vi "UHR-Fleezers Control (host) - 10.6.vi"() -> ()   [LabVIEW 2010] (continued)
            n291 = xnode "Read/Write Control"("FPGA VI Reference In"=w3084, "error in"=w3083, "AI to FIFO"=w3087, "APD to FIFO"=w3087, "Start scan"=w3087, "Start scan (MCL)"=w3087) -> ("FPGA VI Reference Out"=w3089:T20, "error out"=w3088:errorcluster)
          }
        }
        "Raster Scanning..." <- TRUE ("Scanning...")
      }
    }
    n292 = And(x="Save scans", y=w1186) -> (x .and. y?=w1230:bool)
    n293 = Compound Arithmetic op=OR("Start MCL Scan", "Confocal Image", "Confocal Linescan") -> (w1184:bool)
    n294 = And(x="Save Data (MCL)", y=w1184) -> (x .and. y?=w1229:bool)
    n295 = case "Start MCL raster scan" shown="False" w1184 {
      tunnel: w1232 -> [w2240 w2255]
      tunnel: w1231 -> [w2239 w2254]
      tunnel: [w2240 w2250] -> w991
      tunnel: [w2239 w2249] -> w990
      tunnel: [FALSE w2248] -> w1215
      tunnel: "Start MCL Scan" -> [_ w2243]
      tunnel: "Confocal Image" -> [_ w2242]
      tunnel: "Confocal Linescan" -> [_ _]
      frame False {
      }
      frame True {
        w2248 = TRUE
        n296 = case shown="True" "Restart DMA? (MCL)" {
          tunnel: [w2500 w2502] -> w2253
          tunnel: [w2499 w2501] -> w2252
          tunnel: w2255 -> [w2500 w2505]
          tunnel: w2254 -> [w2499 w2504]
          frame False {
          }
          frame True {
            n297 = call "reset FPGA DMA.vi"("error in"=w2504, "FPGA VI Reference In"=w2505) -> ("error out"=w2501:errorcluster, "FPGA VI Reference Out"=w2502:T20)
            n298 = local write "Overflow (data lost)"(FALSE ("Overflow (data lost)")) -> ()
          }
        }
        n299 = case shown="False" w2243 {
          selector: w2243 -> [_ w2259]
          tunnel: w2242 -> [w2258 _]
          tunnel: [w2258 w2259] -> w2241
          frame False {
            n300 = property on="2D or 1D Scan" class="Bool (strict)"("Val(Sgnl)"=w2258) -> ()  [unwired: 2 in, 2 out]
            n301 = property on="Confocal Image" class="Bool (strict)"("Value"=FALSE ("Start Confocal Map")) -> ()  [unwired: 2 in, 2 out]
          }
          frame True {
          }
        }
        n302 = local write "MCL Scanning"(w2248) -> ()
        n303 = local read "AO1"() -> (w2245:dbl)
        n304 = local read "AO2"() -> (w2244:dbl)
        n305 = case shown="True" "Center Scan" {
          tunnel: w2253 -> [w2266 w2378]
          tunnel: w2252 -> [w2265 w2377]
          tunnel: [w2264 w2376] -> w2250
          tunnel: [w2263 w2375] -> w2249
          tunnel: [w2261 w2362] -> w2247
          tunnel: [w2260 w2361] -> w2246
          tunnel: w2245 -> [w2261 w2367]
          tunnel: w2244 -> [w2260 w2370]
          tunnel: w2241 -> [_ _]
          frame False {
            w2262 = TRUE ("AI to FIFO")
            n306 = xnode "Read/Write Control"("FPGA VI Reference In"=w2266, "error in"=w2265, "AI to FIFO"=w2262, "APD to FIFO"=w2262, "Start scan (MCL)"=w2262) -> ("FPGA VI Reference Out"=w2264:T20, "error out"=w2263:errorcluster)
          }
          frame True {
            w2374 = TRUE ("AI to FIFO")
            n307 = local read "Scan steps (MCL)"() -> (w2353:u64)
            n308 = local read "Scan lines (y)"() -> (w2349:u64)
            n309 = local read "Fast Scan Dir"() -> (w2360:bool)
            n310 = local read "Actual MCL Inc (V)"() -> (w2350:dbl)
            n311 = Decrement(x=w2349) -> (x-1=w2348:u64)
            n312 = Decrement(x=w2353) -> (x-1=w2352:u64)
            n313 = Multiply(x=w2350, y=w2348) -> (x*y=w2347:dbl)
            n314 = Divide(x=w2347, y=2.0) -> (x/y=w2357:dbl)
            n315 = Multiply(x=w2350, y=w2352) -> (x*y=w2351:dbl)
            n316 = Divide(x=w2351, y=2.0) -> (x/y=w2356:dbl)
            n317 = Select(t=w2356, s=w2360, f=w2357) -> (s? t:f=w2355:dbl)
            n318 = Select(t=w2357, s=w2360, f=w2356) -> (s? t:f=w2359:dbl)
            n319 = Subtract(x=w2367, y=w2359) -> (x-y=w2358:dbl)
            n320 = Subtract(x=w2370, y=w2355) -> (x-y=w2354:dbl)
            n321 = local read "2D or 1D Scan"() -> (w2372:bool)
            n322 = Not(x=w2360) -> (.not. x?=w2366:bool)
            n323 = Not(x=w2372) -> (.not. x?=w2368:bool)
            n324 = And(x=w2360, y=w2368) -> (x .and. y?=w2369:bool)
            n325 = And(x=w2368, y=w2366) -> (x .and. y?=w2371:bool)
            n326 = Select(t=w2370, s=w2371, f=w2354) -> (s? t:f=w2361:dbl)
            n327 = Select(t=w2367, s=w2369, f=w2358) -> (s? t:f=w2362:dbl)
            n328 = call "Volt to I16.vi"("Voltage In"=w2362) -> ("I16 Voltage Out"=w2365:i16)
            n329 = call "Volt to I16.vi"("Voltage In"=w2361) -> ("I16 Voltage Out"=w2364:i16)
            n330 = xnode "Read/Write Control"("FPGA VI Reference In"=w2378, "error in"=w2377, "AI to FIFO"=w2374, "APD to FIFO"=w2374, "Start scan (MCL)"=w2374, "AO1"=w2365, "AO2"=w2364) -> ("FPGA VI Reference Out"=w2376:T20, "error out"=w2375:errorcluster)
          }
        }
        "Initial Y" <- w2247
        "Initial X" <- w2246
        "wait to reset values" <- w2248
      }
    }
    n331 = local read "Trap Pos Elements/DMA read"() -> (w1065:u32)
    n332 = local read "Trap AI Elements/DMA read"() -> (w989:u32)
    n333 = local read "APD Elements/DMA read"() -> (w1108:u32)
    n334 = local read "Trap AI FIFO Depth"() -> (w1279:u32)
    n335 = xnode "Invoke Method"("FPGA VI Reference In"=w991, "error in"=w990, "Number of Elements"=w1065, "Timeout (ms)"=-1) -> ("Data"=w1029:u16[], "Elements Remaining"=→"Trap Pos FIFO El Remaining":u32)  [unwired: 2 out]
    n336 = xnode "Invoke Method"("FPGA VI Reference In"=w991, "error in"=w990, "Number of Elements"=w989, "Timeout (ms)"=-1 ("Timeout")) -> ("FPGA VI Reference Out"=w993:T20, "error out"=w992:errorcluster, "Data"=w988:i16[], "Elements Remaining"=w994:u32)
    "Trap AI FIFO El. Rem." <- w994
    n337 = xnode "Get APD Data"("FPGA VI Reference In"=w991, "error in"=w990, "Number of Elements"=w1108, "Timeout (ms)"=-1) -> ("Data"=w1107:u32[], "Elements Remaining"=→"APD FIFO Elements Remaining":u32)  [unwired: 2 out]
    n338 = Subtract(x=w1279, y=w989) -> (x-y=w1278:u32)
    n339 = Decimate 1D Array(w1029) -> (w1026:u16[], w1028:u16[], w1027:u16[])
    n340 = Divide(x=w994, y=w1278) -> (x/y=w1277:dbl)
    "Buffer Status" <- w1277
    n341 = To Unsigned Long Integer(number=w1026) -> (unsigned 32bit integer=w1025:u32[])
    n342 = Join Numbers(hi=w1028, lo=w1027) -> ((hi.lo)=w1024:u32[])
    n343 = Equal?(x=w1277, y=1.0) -> (x = y?=w1275:bool)
    n344 = Join Numbers(hi=w1025, lo=w1024) -> ((hi.lo)=w1018:u64[])
    n345 = call "IR AOM word to freq - vec.vi"("Frequency Word In (double vec)"=w1018) -> ("Frequency Out"=w1064:dbl[])
    n346 = case "Alert buffer overflow" shown="True" w1275 {
      frame False {
      }
      frame True {
        n347 = call <vilib>:"Beep.vi"() -> ()  [unwired: 3 in, 9 out]
        "Overflow (data lost)" <- TRUE ("Overflow (data lost)")
      }
    }
    n348 = Decimate 1D Array(w1064) -> (w1063:dbl[], w1062:dbl[])
    n349 = Array Size(array=w988) -> (size(s)=→"Waveform Chart":i32)
    n350 = Build Array(w1063, w1062) -> (w1061:dbl[][])
    n351 = local read "Trap Sets"() -> (w1145:u32)
    n352 = case "Deinterlace trap data, average down PSD" shown="2" w1145 {
      tunnel: w988 -> [w2535 w2600]
      tunnel: [w2532 w2597] -> w1138
      tunnel: [w2535 w2599] -> w1021
      tunnel: "Detector Type" -> [w2534 w2595]
      tunnel: [w2533 w2598] -> w1137
      tunnel: [w2531 w2596] -> w1250
      frame 1, Default {
        n353 = Divide(x=w2535, y=3276.7) -> (x/y=w2536:dbl[])
        n354 = Decimate 1D Array(w2536) -> (w2545:dbl[], w2544:dbl[], w2543:dbl[], w2542:dbl[], w2541:dbl[], w2540:dbl[], w2539:dbl[], w2538:dbl[])
        n355 = case shown="\"IR-QPD + PSD + FB-QPD position\"" w2534 {
          tunnel: w2545 -> [w2569 w2594]
          tunnel: w2544 -> [w2568 w2593]
          tunnel: w2543 -> [w2553 w2571]
          tunnel: w2542 -> [w2554 w2581]
          tunnel: w2541 -> [w2567 w2592]
          tunnel: w2540 -> [w2566 w2591]
          tunnel: w2539 -> [w2550 w2572]
          tunnel: w2538 -> [w2549 w2570]
          tunnel: [w2548 w2578] -> w2533
          tunnel: [w2547 w2577] -> w2532
          tunnel: [w2546 w2576] -> w2531
          frame "IR-QPD + PSD + FB-QPD", Default {
            w2546 = 0  # Channel pattern
            n356 = Divide(x=w2569, y=w2554) -> (x/y=w2556:dbl[])
            n357 = Divide(x=w2568, y=w2554) -> (x/y=w2555:dbl[])
            n358 = Divide(x=w2567, y=w2550) -> (x/y=w2552:dbl[])
            n359 = Divide(x=w2566, y=w2549) -> (x/y=w2551:dbl[])
            n360 = Build Array(w2556, w2555, w2554, w2553, w2552, w2551, w2550, w2549) -> (w2547:dbl[][])
            n361 = Bundle("T1 Y", "T1 X", "T1 Sum", "FB Sum", "PSD Y", "PSD X", "PSD Y Sum", "PSD X Sum") -> (w2565:T40)  [unwired: 1 out]
            n362 = Cluster To Array(cluster=w2565) -> (array=w2548:string[])
          }
          frame "IR-QPD + PSD + FB-QPD position" {
            w2576 = 3  # Channel pattern
            n363 = Negate(x=w2572) -> (-x=w2573:dbl[])
            n364 = Divide(x=w2594, y=w2581) -> (x/y=w2583:dbl[])
            n365 = Divide(x=w2593, y=w2581) -> (x/y=w2582:dbl[])
            n366 = Divide(x=w2592, y=w2572) -> (x/y=w2580:dbl[])
            n367 = Divide(x=w2591, y=w2573) -> (x/y=w2579:dbl[])
            n368 = Build Array(w2583, w2582, w2581, w2570, w2571, w2580, w2579, w2572) -> (w2577:dbl[][])
            n369 = Bundle("T1 Y", "T1 X", "T1 Sum", "FB X", "FB Sum", "PSD Y", "PSD X", "PSD Y Sum") -> (w2590:T40)  [unwired: 1 out]
            n370 = Cluster To Array(cluster=w2590) -> (array=w2578:string[])
          }
        }
      }
      frame 2 {
        n371 = case shown="\"UCB Fleezers 052511\"" w2595 {
          tunnel: w2600 -> [w2662 w2729 w2757 w2864]
          tunnel: [w2601 w2721 w2752 w2795] -> w2599
          tunnel: [w2628 w2712 w2754 w2842] -> w2598
          tunnel: [w2627 w2676 w2731 w2809] -> w2597
          tunnel: [w2621 w2711 w2794 w2840] -> w2596
          frame "IR-QPD + PSD + FB-QPD", Default {
            w2621 = 1  # Channel pattern
            # "time average x2 the 4th signal and the 4 psd signals (detection laser)"
            # "deinterlace 3 signals from qpd"
            n372 = Decimate 1D Array(w2662) -> (w2661:i16[], w2660:i16[], w2626:i16[], w2659:i16[], w2649:i16[], w2647:i16[], w2646:i16[], w2644:i16[])
            n373 = call "downsample 1D array - double.vi"("Ave N"=2.0, "Array In"=w2649) -> ("Array Out"=w2648:dbl[])  [unwired: 1 out]
            n374 = call "downsample 1D array - double.vi"("Ave N"=2.0, "Array In"=w2644) -> ("Array Out"=w2643:dbl[])  [unwired: 1 out]
            n375 = call "downsample 1D array - double.vi"("Ave N"=2.0, "Array In"=w2646) -> ("Array Out"=w2645:dbl[])  [unwired: 1 out]
            n376 = call "downsample 1D array - double.vi"("Ave N"=2.0, "Array In"=w2647) -> ("Array Out"=w2629:dbl[])  [unwired: 1 out]
            n377 = Decimate 1D Array(w2661) -> (w2658:i16[], w2630:i16[])
            n378 = Decimate 1D Array(w2660) -> (w2657:i16[], w2655:i16[])
            n379 = Decimate 1D Array(w2659) -> (w2656:i16[], w2654:i16[])
            n380 = Decimate 1D Array(w2626) -> (w2625:i16[], w2624:i16[])
            n381 = Interleave 1D Arrays(w2658, w2657, w2656, w2630, w2655, w2654, w2625, w2624, w2648, w2629, w2645, w2643) -> (w2642:dbl[])
            n382 = To Word Integer(number=w2642) -> (16bit integer=w2601:i16[])
            n383 = Divide(x=w2642, y=3276.7) -> (x/y=w2641:dbl[])
            n384 = Decimate 1D Array(w2641) -> (w2640:dbl[], w2639:dbl[], w2638:dbl[], w2637:dbl[], w2636:dbl[], w2635:dbl[], w2623:dbl[], w2622:dbl[], w2634:dbl[], w2633:dbl[], w2632:dbl[], w2631:dbl[])
            n385 = Divide(x=w2640, y=w2638) -> (x/y=w2608:dbl[])
            n386 = Divide(x=w2639, y=w2638) -> (x/y=w2607:dbl[])
            n387 = Divide(x=w2637, y=w2635) -> (x/y=w2606:dbl[])
            n388 = Divide(x=w2636, y=w2635) -> (x/y=w2605:dbl[])
            n389 = Divide(x=w2634, y=w2632) -> (x/y=w2604:dbl[])
            n390 = Divide(x=w2633, y=w2631) -> (x/y=w2603:dbl[])
            n391 = Bundle("T1 Y", "T1 X", "T1 Sum", "T2 Y", "T2 X", "T2 Sum", "T1 FB Sum", "T2 FB Sum", "PSD Y", "PSD X", "PSD Y Sum", "PSD X Sum") -> (w2609:T41)  [unwired: 1 out]
            n392 = Build Array(w2608, w2607, w2638, w2606, w2605, w2635, w2623, w2622, w2604, w2603, w2632, w2631) -> (w2627:dbl[][])
            n393 = Cluster To Array(cluster=w2609) -> (array=w2628:string[])
          }
          frame "IR-QPD + PSD + FB-QPD X position" {
            w2711 = 2  # Channel pattern
            # "convert\nADC numbers\nto volts"
            # "time average x2 the 3 psd signals (detection laser)"
            # "deinterlace 3 signals from qpds"
            n394 = Decimate 1D Array(w2729) -> (w2728:i16[], w2727:i16[], w2664:i16[], w2665:i16[], w2674:i16[], w2671:i16[], w2668:i16[], w2699:i16[])
            n395 = Decimate 1D Array(w2728) -> (w2726:i16[], w2713:i16[])
            n396 = call "downsample 1D array - I16.vi"("Ave N"=2.0, "Array In"=w2674) -> ("Array Out"=w2672:i16[])  [unwired: 1 in]
            n397 = call "downsample 1D array - I16.vi"("Ave N"=2.0, "Array In"=w2671) -> ("Array Out"=w2669:i16[])  [unwired: 1 in]
            n398 = Decimate 1D Array(w2727) -> (w2725:i16[], w2723:i16[])
            n399 = Decimate 1D Array(w2665) -> (w2724:i16[], w2722:i16[])
            n400 = Decimate 1D Array(w2699) -> (w2698:i16[], w2696:i16[])
            n401 = Decimate 1D Array(w2664) -> (w2697:i16[], w2695:i16[])
            n402 = call "downsample 1D array - I16.vi"("Ave N"=2.0, "Array In"=w2668) -> ("Array Out"=w2666:i16[])  [unwired: 1 in]
            n403 = Interleave 1D Arrays(w2726, w2725, w2724, w2713, w2723, w2722, w2698, w2697, w2696, w2695, w2672, w2669, w2666) -> (w2721:i16[])
            n404 = Divide(x=w2721, y=3276.7) -> (x/y=w2720:dbl[])
            n405 = Decimate 1D Array(w2720) -> (w2719:dbl[], w2718:dbl[], w2717:dbl[], w2716:dbl[], w2715:dbl[], w2714:dbl[], w2687:dbl[], w2685:dbl[], w2684:dbl[], w2682:dbl[], w2681:dbl[], w2680:dbl[], w2677:dbl[])
            n406 = Divide(x=w2719, y=w2717) -> (x/y=w2703:dbl[])
            n407 = Divide(x=w2718, y=w2717) -> (x/y=w2702:dbl[])
            n408 = Divide(x=w2716, y=w2714) -> (x/y=w2701:dbl[])
            n409 = Divide(x=w2715, y=w2714) -> (x/y=w2700:dbl[])
            n410 = Divide(x=w2687, y=w2685) -> (x/y=w2686:dbl[])
            n411 = Divide(x=w2684, y=w2682) -> (x/y=w2683:dbl[])
            n412 = Divide(x=w2681, y=w2677) -> (x/y=w2679:dbl[])
            n413 = Negate(x=w2677) -> (-x=w2675:dbl[])
            n414 = Divide(x=w2680, y=w2675) -> (x/y=w2678:dbl[])
            n415 = Bundle("T1 Y", "T1 X", "T1 Sum", "T2 Y", "T2 X", "T2 Sum", "T1 FB X", "T1 FB Sum", "T2 FB X", "T2 FB Sum", "PSD Y", "PSD X", "PSD Y Sum") -> (w2704:T42)  [unwired: 1 out]
            n416 = Build Array(w2703, w2702, w2717, w2701, w2700, w2714, w2686, w2685, w2683, w2682, w2679, w2678, w2677) -> (w2676:dbl[][])
            n417 = Cluster To Array(cluster=w2704) -> (array=w2712:string[])
          }
          frame "UCB Fleezers 052511" {
            w2794 = 2  # Channel pattern
            n418 = Decimate 1D Array(w2757) -> (w2792:i16[], w2791:i16[], w2756:i16[], w2755:i16[], w2749:i16[], w2746:i16[], w2745:i16[], w2744:i16[])
            n419 = Decimate 1D Array(w2792) -> (w2790:i16[], w2775:i16[])
            n420 = Decimate 1D Array(w2791) -> (w2789:i16[], w2787:i16[])
            n421 = Decimate 1D Array(w2756) -> (w2788:i16[], w2786:i16[])
            n422 = Decimate 1D Array(w2755) -> (w2751:i16[], w2750:i16[])
            n423 = Decimate 1D Array(w2749) -> (w2748:i16[], w2747:i16[])
            n424 = call "downsample 1D array - I16.vi"("Ave N"=2.0, "Array In"=w2746) -> ("Array Out"=w2743:i16[])  [unwired: 1 in]
            n425 = call "downsample 1D array - I16.vi"("Ave N"=2.0, "Array In"=w2745) -> ("Array Out"=w2742:i16[])  [unwired: 1 in]
            n426 = call "downsample 1D array - I16.vi"("Ave N"=2.0, "Array In"=w2744) -> ("Array Out"=w2741:i16[])  [unwired: 1 in]
            n427 = Interleave 1D Arrays(w2790, w2789, w2788, w2775, w2787, w2786, w2751, w2748, w2750, w2747, w2743, w2742, w2741) -> (w2752:i16[])
            n428 = Divide(x=w2752, y=3276.7) -> (x/y=w2782:dbl[])
            n429 = Decimate 1D Array(w2782) -> (w2781:dbl[], w2780:dbl[], w2779:dbl[], w2778:dbl[], w2777:dbl[], w2776:dbl[], w2740:dbl[], w2738:dbl[], w2737:dbl[], w2735:dbl[], w2734:dbl[], w2733:dbl[], w2732:dbl[])
            n430 = Divide(x=w2781, y=w2779) -> (x/y=w2762:dbl[])
            n431 = Divide(x=w2780, y=w2779) -> (x/y=w2761:dbl[])
            n432 = Divide(x=w2778, y=w2776) -> (x/y=w2760:dbl[])
            n433 = Divide(x=w2777, y=w2776) -> (x/y=w2759:dbl[])
            n434 = Divide(x=w2740, y=w2738) -> (x/y=w2739:dbl[])
            n435 = Divide(x=w2737, y=w2735) -> (x/y=w2736:dbl[])
            n436 = Bundle("T1 Y", "T1 X", "T1 Sum", "T2 Y", "T2 X", "T2 Sum", "T1 FB X", "T2 FB Sum", "T2 FB X", "T2 FB Sum", "PSD Y", "PSD X", "PSD Sum") -> (w2763:T42)  [unwired: 1 out]
            n437 = Build Array(w2762, w2761, w2779, w2760, w2759, w2776, w2739, w2738, w2736, w2735, w2734, w2733, w2732) -> (w2731:dbl[][])
            n438 = Cluster To Array(cluster=w2763) -> (array=w2754:string[])
          }
          frame "IR-QPD + PSD + FB-QPD XY positions" {
            w2840 = 4  # Channel pattern
            # "time average x2 the 3 psd signals (detection laser)"
            # "deinterlace 3 signals from qpds"
            n439 = Decimate 1D Array(w2864) -> (w2863:i16[], w2862:i16[], w2841:i16[], w2861:i16[], w2807:i16[], w2853:i16[], w2852:i16[], w2829:i16[])
            n440 = Decimate 1D Array "QPD Y"(w2863) -> (w2860:i16[], w2843:i16[])
            n441 = call "downsample 1D array - double.vi"("Ave N"=2.0, "Array In"=w2853) -> ("Array Out"=w2828:dbl[])  [unwired: 1 out]
            n442 = call "downsample 1D array - double.vi"("Ave N"=2.0, "Array In"=w2852) -> ("Array Out"=w2827:dbl[])  [unwired: 1 out]
            n443 = Decimate 1D Array "Feedback Sum"(w2841) -> (w2825:i16[], w2823:i16[])
            n444 = Decimate 1D Array "Feedback Y"(w2807) -> (w2806:i16[], w2805:i16[])
            n445 = Decimate 1D Array "Feedback X"(w2829) -> (w2826:i16[], w2824:i16[])
            n446 = Decimate 1D Array "QPD Sum"(w2861) -> (w2858:i16[], w2856:i16[])
            n447 = Decimate 1D Array "QPD X"(w2862) -> (w2859:i16[], w2857:i16[])
            n448 = Interleave 1D Arrays(w2860, w2859, w2858, w2843, w2857, w2856, w2806, w2826, w2825, w2805, w2824, w2823, w2828, w2827) -> (w2851:dbl[])
            n449 = To Word Integer(number=w2851) -> (16bit integer=w2795:i16[])
            n450 = Divide(x=w2851, y=3276.7) -> (x/y=w2850:dbl[])
            n451 = Decimate 1D Array(w2850) -> (w2849:dbl[], w2848:dbl[], w2847:dbl[], w2846:dbl[], w2845:dbl[], w2844:dbl[], w2802:dbl[], w2816:dbl[], w2800:dbl[], w2801:dbl[], w2814:dbl[], w2798:dbl[], w2812:dbl[], w2810:dbl[])
            n452 = Divide(x=w2849, y=w2847) -> (x/y=w2833:dbl[])
            n453 = Divide(x=w2848, y=w2847) -> (x/y=w2832:dbl[])
            n454 = Divide(x=w2846, y=w2844) -> (x/y=w2831:dbl[])
            n455 = Divide(x=w2845, y=w2844) -> (x/y=w2830:dbl[])
            n456 = Divide(x=w2802, y=w2800) -> (x/y=w2799:dbl[])
            n457 = Divide(x=w2816, y=w2800) -> (x/y=w2815:dbl[])
            n458 = Divide(x=w2801, y=w2798) -> (x/y=w2797:dbl[])
            n459 = Divide(x=w2814, y=w2798) -> (x/y=w2813:dbl[])
            n460 = Negate(x=w2810) -> (-x=w2808:dbl[])
            n461 = Divide(x=w2812, y=w2808) -> (x/y=w2811:dbl[])
            n462 = Bundle("T1 Y", "T1 X", "T1 Sum", "T2 Y", "T2 X", "T2 Sum", "T1 FB Y", "T1 FB X", "T1 FB Sum", "T2 FB Y", "T2 FB X", "T2 FB Sum", "PSD X", "PSD Y Sum") -> (w2796:T43)  [unwired: 1 out]
            n463 = Build Array(w2833, w2832, w2847, w2831, w2830, w2844, w2799, w2815, w2800, w2797, w2813, w2798, w2811, w2810) -> (w2809:dbl[][])
            n464 = Cluster To Array(cluster=w2796) -> (array=w2842:string[])
          }
        }
      }
    }
    "AI labels" <- w1137
    n465 = Decimate 1D Array(w1107) -> (w1135:u32[], w1071:u32[])
    n466 = local read "DMA Update Period (s)"() -> (w1146:dbl)
    n467 = local read "BD 1 Frequency 2 (MHz)"() -> (w1013:dbl)
    n468 = local read "BD 1 Frequency 1 (MHz)"() -> (w1014:dbl)
    n469 = Build Array(w1135, w1071) -> (w1212:u32[][])
    n470 = local read "Data Period (s)"() -> (w1120:dbl)
    n471 = Decimate 1D Array(w1021) -> (w1044:i16[], w1043:i16[], w1041:i16[], w1040:i16[])  [unwired: 9 out]
    n472 = To Double Precision Float(number=w1212) -> (double precision float=w1213:dbl[][])
    n473 = local read "APD Integration Time (s)"() -> (w1084:dbl)
    n474 = Divide(x=w1044, y=w1043) -> (x/y=w1045:dbl[])
    n475 = Divide(x=w1041, y=w1040) -> (x/y=w1042:dbl[])
    n476 = feedback #1(0.0) -> (w1058:dbl)
    n477 = Add(x=w1146, y=w1058) -> (x+y=w1252:dbl)
    n478 = feedback-in #1(w1252) -> ()
    n479 = local read "AOM X Cal (nm/MHz)"() -> (w1011:dbl)
    n480 = To Time Stamp(1:w1058) -> (0:w1057:timestamp)
    n481 = Split 1D Array(array=w1045, index="N El. to Ave.") -> (second subarray=w1048:dbl[])  [unwired: 1 out]
    n482 = Split 1D Array(array=w1042, index="N El. to Ave.") -> (second subarray=w1047:dbl[])  [unwired: 1 out]
    n483 = local read "Trap X AI1 (DMA)"() -> (w1046:T13)
    n484 = Multiply(x=w1120, y="Trap Disp. Downsample") -> (x*y=w1059:dbl)
    "Display Period (s)" <- w1059
    n485 = Bundle("BD 1 Frequency 1 (MHz)"=w1014, "BD 1 Frequency 2 (MHz)"=w1013) -> (w1015:T44)  [unwired: 1 out]
    n486 = for "Trap AI" {
      tunnel: [w2530] -> w1246 mode=indexing
      tunnel: w1057 -> [w2520]
      tunnel: "Trap Disp. Downsample" -> [w2528]
      tunnel: w1138 -> [w2526] mode=indexing
      tunnel: w1120 -> [w2525]
      tunnel: w1137 -> [w2524] mode=indexing
      tunnel: w1056 -> [w2523]
      tunnel: [w2522] -> w1095 mode=indexing
      tunnel: w1059 -> [w2521]
      n487 = Bundle By Name("Y"=w2526, "dt"=w2525) -> (w2527:waveform(dbl))  [unwired: 1 out]
      n488 = Set Waveform Attribute(5:w2524, 6:w2523, 7:w2527) -> (3:w2522:waveform(dbl))  [unwired: 1 in, 2 out]
      n489 = call "downsample 1D array - double.vi"("Ave N"=w2528, "Array In"=w2526) -> ("Array Out"=w2529:dbl[])  [unwired: 1 out]
      n490 = Bundle By Name(cluster=w2522, "t0"=w2520, "Y"=w2529, "dt"=w2521) -> (w2530:waveform(dbl))
    }
    n491 = call <vilib>:"Mean.vi"("X"=w1047) -> ("mean"=w1035:dbl)  [unwired: 1 out]
    n492 = call <vilib>:"Mean.vi"("X"=w1048) -> ("mean"=w1036:dbl)  [unwired: 1 out]
    n493 = Cluster To Array(cluster=w1015) -> (array=w1012:dbl[])
    n494 = Reciprocal(x=w1059) -> (1/x=→"Trap Disp. Freq. (Hz)":dbl)
    n495 = local read "Data points/scans (MCL)"() -> (w1224:dbl)
    n496 = To Fixed-Point(number=w1035) -> (fixed-point=w1033:fxp<+/-,16,1>)  [unwired: 1 in]
    n497 = To Fixed-Point(number=w1036) -> (fixed-point=w1034:fxp<+/-,16,1>)  [unwired: 1 in]
    n498 = Bundle("Trap 1 Pos.", "Trap 2 Pos.") -> (w1055:cluster{string, string})  [unwired: 1 out]
    n499 = Bundle By Name(cluster=w1046, "Set 1"=w1034, "Set 2"=w1033) -> (→"Trap X AI1 (DMA)":T13)
    n500 = Cluster To Array(cluster=w1055) -> (array=w1052:string[])
    n501 = for "Trap Position" {
      tunnel: w1061 -> [w1507] mode=indexing
      tunnel: "Trap Disp. Downsample" -> [w1506]
      tunnel: w1059 -> [w1504]
      tunnel: w1057 -> [w1503]
      tunnel: w1056 -> [w1501]
      tunnel: w1052 -> [w1500] mode=indexing
      tunnel: [w1499] -> w1010 mode=indexing
      tunnel: w1012 -> [w1497] mode=indexing
      tunnel: w1011 -> [w1495]
      n502 = call "downsample 1D array - double.vi"("Ave N"=w1506, "Array In"=w1507) -> ("Array Out"=w1505:dbl[])  [unwired: 1 out]
      n503 = Subtract(x=w1505, y=w1497) -> (x-y=w1498:dbl[])
      n504 = Multiply(x=w1495, y=w1498) -> (x*y=w1496:dbl[])
      n505 = Bundle By Name("Y"=w1496, "dt"=w1504, "t0"=w1503) -> (w1502:waveform(dbl))  [unwired: 1 out]
      n506 = Set Waveform Attribute(5:w1500, 6:w1501, 7:w1502) -> (3:w1499:waveform(dbl))  [unwired: 1 in, 2 out]
    }
    "Trap Positions" <- w1010
    n507 = Bundle("APD 1", "APD 2") -> (w1245:cluster{string, string})  [unwired: 1 out]
    n508 = Cluster To Array(cluster=w1245) -> (array=w1242:string[])
    n509 = for "APD" {
      tunnel: w1213 -> [w2509] mode=indexing
      tunnel: w1084 -> [w2517]
      tunnel: [w2513] -> w1091 mode=indexing
      tunnel: "APD Disp. Scale" -> [w2514]
      tunnel: w1056 -> [w2512]
      tunnel: w1242 -> [w2511] mode=indexing
      tunnel: "APD Disp. Downsample" -> [w2507]
      tunnel: [w2510] -> w1241
      tunnel: w1057 -> [w2506]
      n510 = call "integrate 1D array interval - double.vi"("Ave N"=w2507, "Array In"=w2509) -> ("Array Out"=w2508:dbl[])  [unwired: 1 out]
      n511 = Multiply(x=w2517, y=w2507) -> (x*y=w2510:dbl)
      n512 = Divide(x=w2508, y=w2514) -> (x/y=w2515:dbl[])
      n513 = Bundle By Name("t0"=w2506, "Y"=w2515, "dt"=w2510) -> (w2516:waveform(dbl))  [unwired: 1 out]
      n514 = Set Waveform Attribute(5:w2511, 6:w2512, 7:w2516) -> (3:w2513:waveform(dbl))  [unwired: 1 in, 2 out]
    }
    "APD Display Period (s)" <- w1241
    n515 = Reciprocal(x=w1241) -> (1/x=→"APD Display Freq. (Hz)":dbl)
    n516 = local read "Display Period (s)"() -> (w1119:dbl)
    n517 = Increment(x=w1224) -> (x+1=w1225:dbl)
    n518 = Index Array(array=w1010, index=0) -> (element=w1008:waveform(dbl))
    n519 = To Double Precision Float(number=w1135) -> (double precision float=w1134:dbl[])
    n520 = feedback #2(w1225) -> (w1228:dbl)
    n521 = Select(t=0, s=w1215, f=w1228) -> (s? t:f=w1221:dbl)
    n522 = Array Size(array=w1134) -> (size(s)=w1227:i32)
    n523 = Add(x=w1227, y=w1221) -> (x+y=w1222:dbl)
    n524 = Unbundle By Name(w1008) -> ("Y"=w1006:dbl[])
    n525 = feedback #3(w1135) -> (w1211:u32[])
    n526 = Build Array (concatenate)(w1211, w1135) -> (w1208:u32[])
    n527 = feedback #4(w1071) -> (w1090:u32[])
    n528 = Divide(x="Bead Sep. Int. Time (s)", y=w1119) -> (x/y=w1004:dbl)
    n529 = Build Array (concatenate)(w1090, w1071) -> (w1089:u32[])
    n530 = Greater?(x=w1222, y=w1224) -> (0:w1223:bool)
    n531 = feedback #5(w1006) -> (w1007:dbl[])
    n532 = Build Array (concatenate)(w1006, w1007) -> (w1005:dbl[])
    n533 = Select(t=w1221, s=w1223, f=w1222) -> (s? t:f=w1220:dbl)
    n534 = feedback-in #2(w1220) -> ()
    n535 = Array Size(array=w1208) -> (size(s)=w1205:i32)
    n536 = Array Size(array=w1135) -> (size(s)=w1207:i32)
    n537 = local read "MCL Scanning"() -> (w1218:bool)
    n538 = local read "APD Integration Time (s)"() -> (w1098:dbl)
    n539 = Build Array (concatenate)(w1091, w1246) -> (w1093:waveform(dbl)[])
    "All Signals" <- w1093
    n540 = Split 1D Array(array=w1005, index=w1004) -> (first subarray=w998:dbl[])  [unwired: 1 out]
    n541 = feedback-in #5(w998) -> ()
    n542 = Multiply(x=w1207, y="APD Ave N") -> (x*y=w1206:dbl)
    n543 = Greater?(x=w1205, y=w1206) -> (0:w1209:bool)
    n544 = Not(x=w1223) -> (.not. x?=w1217:bool)
    n545 = To Double Precision Float(number=w1071) -> (double precision float=w1070:dbl[])
    n546 = call <vilib>:"Mean.vi"("X"=w998) -> ("mean"=w997:dbl)  [unwired: 1 out]
    "Mean T1 Position (nm)" <- w997
    n547 = Subtract(x=w998, y=w997) -> (x-y=w1003:dbl[])
    n548 = Square(x=w1003) -> (x^2=w1002:dbl[])
    n549 = And(x=w1217, y=w1218) -> (x .and. y?=w1219:bool)
    n550 = call <vilib>:"Mean.vi"("X"=w1002) -> ("mean"=w1001:dbl)  [unwired: 1 out]
    n551 = case shown="True" w1209 {
      tunnel: w1208 -> [w2090 w2097]
      tunnel: [w2090 w2095] -> w1151
      tunnel: w1206 -> [_ w2092]
      tunnel: w1205 -> [_ w2096]
      tunnel: w1089 -> [w2089 w2094]
      tunnel: [w2089 w2091] -> w1086
      frame False {
      }
      frame True {
        n552 = Subtract(x=w2096, y=w2092) -> (x-y=w2093:dbl)
        n553 = Array Subset(array=w2097, index=w2093, length=w2092) -> (w2095:u32[])
        n554 = Array Subset(array=w2094, index=w2093, length=w2092) -> (w2091:u32[])
      }
    }
    n555 = feedback-in #3(w1151) -> ()
    n556 = feedback-in #4(w1086) -> ()
    n557 = Or(x=w1219, y=w1215) -> (x .or. y?=w1216:bool)
    n558 = Square Root(x=w1001) -> (sqrt(x)=w1000:dbl)
    n559 = Equal?(x="Tab Control 6", y=T32."High Res Display") -> (x = y?=w1141:bool)
    n560 = Multiply(x="APD Disp. Scale", y=w1091) -> (x*y=w1100:waveform(dbl)[])
    n561 = Multiply(x="APD Disp. Downsample", y=w1098) -> (x*y=w1096:dbl)
    n562 = Multiply(x=10.0, y=w1000) -> (x*y=→"Trap 1 Position RMS (A)":dbl)
    n563 = Divide(x=w1100, y=w1096) -> (x/y=w1068:waveform(dbl)[])
    n564 = Index Array(array=w1068, index=0) -> (element=w1078:waveform(dbl))
    n565 = case "For computing FFTs for display" shown="True" "Compute FFT" {
      tunnel: w1095 -> [_ w3417]
      frame False {
      }
      frame True {
        n566 = Build Array("FFT 1 Choice 1", "FFT 1 Choice 2", "FFT 2 Choice 1", "FFT 2 Choice 2") -> (w3410:u16[])
        n567 = Array Size(array=w3417) -> (size(s)=w3416:i32)
        n568 = feedback-in #6(w3410) -> ()
        n569 = feedback #6(u16[] [100, 100, 100, 100]) -> (w3411:u16[])
        n570 = feedback-in #7("# Spectra to Ave.") -> ()
        n571 = feedback #7("# Spectra to Ave.") -> (w3408:dbl)
        n572 = Not Equal?(x="# Spectra to Ave.", y=w3408) -> (x != y?=w3407:bool)
        n573 = Not Equal?(x=w3410, y=w3411) -> (x != y?=w3409:bool)
        n574 = feedback #8(1.0) -> (w3394:dbl)
        n575 = Compound Arithmetic op=OR("Reset FFT", w3409, w3407) -> (w3392:bool)
        n576 = Select(t=1.0, s=w3392, f=w3394) -> (s? t:f=w3396:dbl)
        n577 = Greater?(x=w3396, y="# Spectra to Ave.") -> (0:w3415:bool)
        n578 = Increment(x=w3396) -> (x+1=w3395:dbl)
        n579 = feedback-in #8(w3395) -> ()
        n580 = local read "DMA Update Period (s)"() -> (w3390:dbl)
        n581 = Multiply(x="# Spectra to Ave.", y=w3390) -> (x*y=→"Ave. Time (s)":dbl)
        n582 = Build Array(cluster{"f0":dbl, "df":dbl, "magnitude":dbl[]} {"f0"=0.0, "df"=0.0, "magnitude"=[]} ("PSD")) -> (w3399:cluster{"f0":dbl, "df":dbl, "magnitude":dbl[]}[])
        n583 = Build Array(w3399, w3399, w3399, w3399) -> (w3401:T45)
        n584 = feedback #9(w3401) -> (w3406:T45)
        n585 = for {
          N: 4 -> [_]
          tunnel: w3410 -> [w3439] mode=indexing
          tunnel: w3417 -> [w3440]
          tunnel: w3416 -> [w3442]
          tunnel: w3392 -> [w3435]
          tunnel: w3415 -> [w3434]
          tunnel: "# Spectra to Ave." -> [w3433]
          tunnel: [w3432] -> w3405 mode=indexing
          tunnel: w3406 -> [w3437] mode=indexing
          tunnel: [w3436] -> w3393 mode=indexing
          tunnel: w3396 -> [w3431]
          n586 = Less?(x=w3439, y=w3442) -> (x < y?=w3441:bool)
          n587 = Index Array(array=w3440, index=w3439) -> (element=w3438:waveform(dbl))
          n588 = case shown="True" w3441 {
            tunnel: w3438 -> [_ w3459]
            tunnel: w3437 -> [w3444 w3457]
            tunnel: [w3444 w3445] -> w3436
            tunnel: w3435 -> [_ w3456]
            tunnel: w3434 -> [_ w3449]
            tunnel: w3433 -> [_ w3448]
            tunnel: [cluster{"f0":dbl, "df":dbl, "magnitude":dbl[]} {"f0"=0.0, "df"=0.0, "magnitude"=[]} ("PSD") w3450] -> w3432
            tunnel: w3431 -> [_ w3447]
            frame False {
            }
            frame True {
              n589 = call <vilib>:"Std Deviation and Variance.vi"("X"=w3459) -> ("mean"=w3460:dbl)  [unwired: 1 in, 2 out]
              n590 = Subtract(x=w3459, y=w3460) -> (x-y=w3458:waveform(dbl))
              n591 = xnode "Spectral Measurements"("Signals"=w3458) -> ("PSD"=w3452:cluster{"f0":dbl, "df":dbl, "magnitude":dbl[]})  [unwired: 1 in, 1 out]
              n592 = case shown="False" w3456 {
                tunnel: w3457 -> [w3469 _]
                tunnel: [w3465 w3474] -> w3445
                tunnel: w3452 -> [w3468 w3475]
                tunnel: w3449 -> [w3467 _]
                frame False {
                  n593 = Build Array (concatenate)(w3469, w3468) -> (w3466:cluster{"f0":dbl, "df":dbl, "magnitude":dbl[]}[])
                  n594 = case shown="True" w3467 {
                    tunnel: w3466 -> [w3470 w3473]
                    tunnel: [w3470 w3471] -> w3465
                    frame False {
                    }
                    frame True {
                      n595 = Delete From Array(array=w3473, index=0) -> (array with subset deleted=w3471:cluster{"f0":dbl, "df":dbl, "magnitude":dbl[]}[])  [unwired: 1 in, 1 out]
                    }
                  }
                }
                frame True {
                  n596 = Build Array(w3475) -> (w3474:cluster{"f0":dbl, "df":dbl, "magnitude":dbl[]}[])
                }
              }
              n597 = for {
                tunnel: w3445 -> [w3464] mode=indexing
                tunnel: [w3463] -> w3455 mode=indexing
                workers-P: _ -> [_]
                n598 = Unbundle By Name(w3464) -> ("magnitude"=w3463:dbl[])
              }
              n599 = Transpose 2D Array(2D array=w3455) -> (transposed array=w3454:dbl[][])
              n600 = for {
                tunnel: w3454 -> [w3462] mode=indexing
                tunnel: [w3461] -> w3453 mode=indexing
                workers-P: _ -> [_]
                n601 = Add Array Elements(numeric array=w3462) -> (sum=w3461:dbl)
              }
              n602 = Select(t=w3448, s=w3449, f=w3447) -> (s? t:f=w3446:dbl)
              n603 = Divide(x=w3453, y=w3446) -> (x/y=w3451:dbl[])
              n604 = Bundle By Name(cluster=w3452, "magnitude"=w3451) -> (w3450:cluster{"f0":dbl, "df":dbl, "magnitude":dbl[]})
            }
          }
        }
        n605 = case shown="True" w3392 {
          tunnel: w3393 -> [w3424 w3430]
          tunnel: [w3424 w3425] -> w3391
          frame False {
          }
          frame True {
            n606 = Array Subset(array=w3430, index (row)=0 ("index"), length (row)=4 ("length"), index (col)=0 ("index"), length (col)=1 ("length")) -> (w3425:T45)
          }
        }
        n607 = feedback-in #9(w3391) -> ()
        n608 = Split 1D Array(array=w3405, index=2) -> (first subarray=→"FFT 1":cluster{"f0":dbl, "df":dbl, "magnitude":dbl[]}[], second subarray=→"FFT 2":cluster{"f0":dbl, "df":dbl, "magnitude":dbl[]}[])
      }
    }
    n609 = Index Array(array=w1068, index=1) -> (element=w1076:waveform(dbl))
    n610 = case "For displaying the high resolution display (no downsampling)" shown="True" w1141 {
      tunnel: w1095 -> [_ w1599]
      frame False {
      }
      frame True {
        n611 = Index Array(array=w1599, index="High Res. Display") -> (element=w1600:waveform(dbl))
        n612 = call <vilib>:"Std Deviation and Variance.vi"("X"=w1600) -> ("mean"=w1607:dbl, "standard deviation"=w1612:dbl)  [unwired: 1 in, 1 out]
        "Mean Intensity" <- w1607
        "Sigma" <- w1612
        n613 = Subtract(x=w1600, y=w1607) -> (x-y=w1606:waveform(dbl))
        n614 = Select(t=w1606, s="Subtract mean", f=w1600) -> (s? t:f=→"1 Channel":waveform(dbl))
        n615 = Divide(x=w1612, y=w1607) -> (x/y=→"Sigma/Mean":dbl)
        n616 = feedback #10(1) -> (w1601:i32)
        n617 = Greater Or Equal?(x=w1601, y="Slow mean N ave.") -> (x >= y?=w1614:bool)
        n618 = Increment(x=w1601) -> (x+1=w1616:i32)
        n619 = Select(t=1, s=w1614, f=w1616) -> (s? t:f=w1603:i32)
        n620 = feedback-in #10(w1603) -> ()
        n621 = feedback #11() -> (w1604:waveform(dbl))  [unwired: 1 out]
        n622 = case shown="Default" w1601 {
          tunnel: [w1619 w1622] -> w1605
          tunnel: w1604 -> [w1621 _]
          tunnel: w1600 -> [w1620 w1622]
          frame Default {
            n623 = call-poly <vilib>:"Append Waveforms.vi"("waveform B"=w1620, "waveform A"=w1621) -> ("waveform out"=w1619:waveform(dbl))  [unwired: 1 in, 8 out]
          }
          frame 1 {
          }
        }
        n624 = feedback-in #11(w1605) -> ()
        n625 = case shown="True" w1614 {
          tunnel: w1605 -> [_ w1618]
          frame False {
          }
          frame True {
            n626 = call <vilib>:"Mean.vi"("X"=w1618) -> ("mean"=→"Slow mean":dbl)  [unwired: 1 out]
          }
        }
      }
    }
    n627 = case "For plotting results of scanning MCL" shown="True" w1216 {
      tunnel: w1215 -> [_ w2130]
      tunnel: w1134 -> [_ w2226]
      tunnel: w1224 -> [_ _]
      tunnel: w1095 -> [_ w2200]
      tunnel: w1070 -> [_ w2131]
      tunnel: w1069 -> [_ w2104]
      frame False {
      }
      frame True {
        w2111 = u32 0 items=["Horizontal", "Vertical", "Central", "1st Diagonal", "2nd Diagonal"] ("Type of Symmetry")
        w2139 = u32 0 items=["Horizontal", "Vertical", "Central", "1st Diagonal", "2nd Diagonal"] ("Type of Symmetry")
        w2142 = u32 0 items=["Horizontal", "Vertical", "Central", "1st Diagonal", "2nd Diagonal"] ("Type of Symmetry")
        w2171 = u32 0 items=["Horizontal", "Vertical", "Central", "1st Diagonal", "2nd Diagonal"] ("Type of Symmetry")
        n628 = Index Array(array=w2200, index=10) -> (element=w2206:waveform(dbl))
        n629 = Index Array(array=w2200, index=11) -> (element=w2203:waveform(dbl))
        n630 = local read "Cycles/step (MCL)"() -> (w2156:u64)
        n631 = Index Array(array=w2200, index="Channel") -> (element=w2202:waveform(dbl))
        n632 = Unbundle(w2104) -> ("New Image"=w2103:T2, "New Image"=w2102:T2, "New Image"=w2101:T2, "New Image"=w2100:T2)
        n633 = Unbundle By Name(w2206) -> ("Y"=w2158:dbl[])
        n634 = Unbundle By Name(w2203) -> ("Y"=w2160:dbl[])
        n635 = Unbundle By Name(w2202) -> ("Y"=w2165:dbl[])
        n636 = call "downsample 1D array - double.vi"("Ave N"=w2156, "Array In"=w2158) -> ("Array Out"=w2157:dbl[])  [unwired: 1 out]
        n637 = call "downsample 1D array - double.vi"("Ave N"=w2156, "Array In"=w2160) -> ("Array Out"=w2159:dbl[])  [unwired: 1 out]
        n638 = call "downsample 1D array - double.vi"("Ave N"=w2156, "Array In"=w2165) -> ("Array Out"=w2164:dbl[])  [unwired: 1 out]
        n639 = feedback #12(w2226) -> (w2227:dbl[])
        n640 = Build Array (concatenate)(w2227, w2226) -> (w2208:dbl[])
        n641 = feedback #13(w2131) -> (w2133:dbl[])
        n642 = Build Array (concatenate)(w2133, w2131) -> (w2132:dbl[])
        n643 = local read "Scan steps (MCL)"() -> (w2113:u64)
        n644 = Select(t=w2226, s=w2130, f=w2208) -> (s? t:f=w2212:dbl[])
        n645 = feedback-in #12(w2212) -> ()
        n646 = Select(t=w2131, s=w2130, f=w2132) -> (s? t:f=w2114:dbl[])
        n647 = feedback-in #13(w2114) -> ()
        n648 = local read "Scan lines (y)"() -> (w2099:u64)
        n649 = local read "N APD Samp/step"() -> (w2115:dbl)
        n650 = feedback #14(w2157) -> (w2214:dbl[])
        n651 = Build Array (concatenate)(w2214, w2157) -> (w2205:dbl[])
        n652 = feedback #15(w2164) -> (w2224:dbl[])
        n653 = Build Array (concatenate)(w2224, w2164) -> (w2223:dbl[])
        n654 = feedback #16(w2159) -> (w2216:dbl[])
        n655 = Build Array (concatenate)(w2216, w2159) -> (w2217:dbl[])
        n656 = Select(t=w2157, s=w2130, f=w2205) -> (s? t:f=w2161:dbl[])
        n657 = feedback-in #14(w2161) -> ()
        n658 = Select(t=w2164, s=w2130, f=w2223) -> (s? t:f=w2163:dbl[])
        n659 = feedback-in #15(w2163) -> ()
        n660 = Select(t=w2159, s=w2130, f=w2217) -> (s? t:f=w2162:dbl[])
        n661 = feedback-in #16(w2162) -> ()
        n662 = Multiply(x=w2113, y=u64 2) -> (x*y=w2098:u64)
        n663 = call "integrate 1D array interval - double.vi"("Ave N"=w2115, "Array In"=w2114) -> ("Array Out"=w2126:dbl[])  [unwired: 1 out]
        n664 = call "integrate 1D array interval - double.vi"("Ave N"=w2115, "Array In"=w2212) -> ("Array Out"=w2211:dbl[])  [unwired: 1 out]
        n665 = Array Size(array=w2126) -> (size(s)=w2127:i32)
        n666 = Array Size(array=w2211) -> (size(s)=w2213:i32)
        n667 = Multiply(x=w2099, y=w2098) -> (x*y=w2129:u64)
        n668 = Multiply(x=w2099, y=w2098) -> (x*y=w2221:u64)
        n669 = call <vilib>:"Mean.vi"("X"=w2161) -> ("mean"=w2145:dbl)  [unwired: 1 out]
        n670 = Subtract(x=w2129, y=w2127) -> (x-y=w2120:u64)
        n671 = call <vilib>:"Mean.vi"("X"=w2163) -> ("mean"=w2150:dbl)  [unwired: 1 out]
        n672 = call <vilib>:"Mean.vi"("X"=w2162) -> ("mean"=w2148:dbl)  [unwired: 1 out]
        n673 = call <vilib>:"Mean.vi"("X"=w2126) -> ("mean"=w2117:dbl)  [unwired: 1 out]
        n674 = Subtract(x=w2221, y=w2213) -> (x-y=w2155:u64)
        n675 = call <vilib>:"Mean.vi"("X"=w2211) -> ("mean"=w2152:dbl)  [unwired: 1 out]
        n676 = Initialize Array(1.0 ("element"), w2120) -> (w2116:dbl[])
        n677 = Initialize Array(1.0 ("element"), w2155) -> (w2146:dbl[])
        n678 = Multiply(x=w2116, y=w2117) -> (x*y=w2118:dbl[])
        n679 = Multiply(x=w2146, y=w2148) -> (x*y=w2149:dbl[])
        n680 = Multiply(x=w2146, y=w2150) -> (x*y=w2151:dbl[])
        n681 = Multiply(x=w2146, y=w2145) -> (x*y=w2147:dbl[])
        n682 = Multiply(x=w2146, y=w2152) -> (x*y=w2153:dbl[])
        n683 = Build Array (concatenate)(w2161, w2147) -> (w2215:dbl[])
        n684 = Build Array (concatenate)(w2163, w2151) -> (w2219:dbl[])
        n685 = Build Array (concatenate)(w2162, w2149) -> (w2218:dbl[])
        n686 = Build Array (concatenate)(w2126, w2118) -> (w2128:dbl[])
        n687 = Build Array (concatenate)(w2211, w2153) -> (w2220:dbl[])
        n688 = Reshape Array(w2215, w2099, w2098) -> (w2181:dbl[][])
        n689 = Reshape Array(w2128, w2099, w2098) -> (w2124:dbl[][])
        n690 = Reshape Array(w2219, w2099, w2098) -> (w2173:dbl[][])
        n691 = Reshape Array(w2218, w2099, w2098) -> (w2188:dbl[][])
        n692 = Reshape Array(w2220, w2099, w2098) -> (w2198:dbl[][])
        n693 = Array Subset(array=w2188, index (col)=0 ("index"), length (col)=w2113) -> (w2193:dbl[][])  [unwired: 2 in]
        n694 = Array Subset(array=w2188, index (col)=w2113) -> (w2191:dbl[][])  [unwired: 3 in]
        n695 = Array Subset(array=w2173, index (col)=0 ("index"), length (col)=w2113) -> (w2179:dbl[][])  [unwired: 2 in]
        n696 = Array Subset(array=w2173, index (col)=w2113) -> (w2177:dbl[][])  [unwired: 3 in]
        n697 = Array Subset(array=w2124, index (col)=0 ("index"), length (col)=w2113) -> (w2123:dbl[][])  [unwired: 2 in]
        n698 = Array Subset(array=w2124, index (col)=w2113) -> (w2121:dbl[][])  [unwired: 3 in]
        n699 = Array Subset(array=w2198, index (col)=0 ("index"), length (col)=w2113) -> (w2197:dbl[][])  [unwired: 2 in]
        n700 = Array Subset(array=w2198, index (col)=w2113) -> (w2195:dbl[][])  [unwired: 3 in]
        n701 = Array Subset(array=w2181, index (col)=0 ("index"), length (col)=w2113) -> (w2186:dbl[][])  [unwired: 2 in]
        n702 = Array Subset(array=w2181, index (col)=w2113) -> (w2184:dbl[][])  [unwired: 3 in]
        n703 = for {
          tunnel: w2193 -> [w2235] mode=indexing
          tunnel: [w2234] -> w2192 mode=indexing
          workers-P: _ -> [_]
          n704 = Reverse 1D Array(array=w2235) -> (reversed array=w2234:dbl[])
        }
        n705 = for {
          tunnel: w2179 -> [w2231] mode=indexing
          tunnel: [w2230] -> w2178 mode=indexing
          workers-P: _ -> [_]
          n706 = Reverse 1D Array(array=w2231) -> (reversed array=w2230:dbl[])
        }
        n707 = for {
          tunnel: w2123 -> [w2229] mode=indexing
          tunnel: [w2228] -> w2122 mode=indexing
          workers-P: _ -> [_]
          n708 = Reverse 1D Array(array=w2229) -> (reversed array=w2228:dbl[])
        }
        n709 = for {
          tunnel: w2197 -> [w2237] mode=indexing
          tunnel: [w2236] -> w2196 mode=indexing
          workers-P: _ -> [_]
          n710 = Reverse 1D Array(array=w2237) -> (reversed array=w2236:dbl[])
        }
        n711 = for {
          tunnel: w2186 -> [w2233] mode=indexing
          tunnel: [w2232] -> w2185 mode=indexing
          workers-P: _ -> [_]
          n712 = Reverse 1D Array(array=w2233) -> (reversed array=w2232:dbl[])
        }
        n713 = Index Array(array=w2198, index (row)=0) -> (element=→"Waveform Graph":dbl[])  [unwired: 1 in]
        n714 = Add(x=w2192, y=w2191) -> (x+y=w2190:dbl[][])
        n715 = Add(x=w2178, y=w2177) -> (x+y=w2176:dbl[][])
        n716 = Add(x=w2122, y=w2121) -> (x+y=w2106:dbl[][])
        n717 = Add(x=w2196, y=w2195) -> (x+y=w2170:dbl[][])
        n718 = Add(x=w2185, y=w2184) -> (x+y=w2183:dbl[][])
        n719 = Divide(x=w2176, y=2) -> (x/y=w2174:dbl[][])
        n720 = Divide(x=w2190, y=2) -> (x/y=w2135:dbl[][])
        n721 = Divide(x=w2183, y=2) -> (x/y=w2137:dbl[][])
        n722 = To Single Precision Float(number=w2170) -> (single precision float=w2169:sgl[][])
        n723 = Transpose 2D Array(2D array=w2174) -> (transposed array=→"Data map":dbl[][])
        n724 = To Single Precision Float(number=w2106) -> (single precision float=w2110:sgl[][])
        n725 = To Single Precision Float(number=w2135) -> (single precision float=w2141:sgl[][])
        n726 = To Single Precision Float(number=w2137) -> (single precision float=w2138:sgl[][])
        n727 = call "IMAQ ArrayToImage"("Image Pixels (Float)"=w2169, "Image"=w2103) -> ("Image Out"=w2172:T2)  [unwired: 8 in, 1 out]
        n728 = call "IMAQ ArrayToImage"("Image Pixels (Float)"=w2110, "Image"=w2102) -> ("Image Out"=w2112:T2)  [unwired: 8 in, 1 out]
        n729 = call "IMAQ ArrayToImage"("Image Pixels (Float)"=w2141, "Image"=w2101) -> ("Image Out"=w2143:T2)  [unwired: 8 in, 1 out]
        n730 = call "IMAQ ArrayToImage"("Image Pixels (Float)"=w2138, "Image"=w2100) -> ("Image Out"=w2140:T2)  [unwired: 8 in, 1 out]
        n731 = call "IMAQ Symmetry"("Type of Symmetry"=w2171, "Image Src"=w2172) -> ("Image Dst Out"=w2167:T2)  [unwired: 3 in, 1 out]
        n732 = call "IMAQ Symmetry"("Type of Symmetry"=w2111, "Image Src"=w2112) -> ("Image Dst Out"=w2108:T2)  [unwired: 3 in, 1 out]
        n733 = call "IMAQ Symmetry"("Type of Symmetry"=w2142, "Image Src"=w2143) -> ("Image Dst Out"=→"Detection Laser X":T2)  [unwired: 3 in, 1 out]
        n734 = call "IMAQ Symmetry"("Type of Symmetry"=w2139, "Image Src"=w2140) -> ("Image Dst Out"=→"Detection Laser Y":T2)  [unwired: 3 in, 1 out]
        n735 = call "IMAQ Set Simple Calibration"("Calibration Axis Info"=T33 {"Origin Pixel"={"X"=0.0, "Y"=0.0}, "Angle Relative to Horizontal (deg)"=0.0, "Axis Reference"=0}, "Grid Descriptor"=T34 {"X Step"=0.3, "Y Step"=0.3, "Unit"=enum."Undefined"}, "Image"=w2167) -> ("Calibrated Image"=→"APD 1":T2)  [unwired: 7 in, 1 out]
        n736 = call "IMAQ Set Simple Calibration"("Calibration Axis Info"=T33 {"Origin Pixel"={"X"=0.0, "Y"=0.0}, "Angle Relative to Horizontal (deg)"=0.0, "Axis Reference"=0}, "Grid Descriptor"=T34 {"X Step"=0.3, "Y Step"=0.3, "Unit"=enum."Undefined"}, "Image"=w2108) -> ("Calibrated Image"=→"APD 2":T2)  [unwired: 7 in, 1 out]
      }
    }
    n737 = Subtract(x=w1076, y="APD 2 Offset") -> (x-y=w1073:waveform(dbl))
    n738 = Subtract(x=w1078, y="APD 1 Offset") -> (x-y=w1074:waveform(dbl))
    n739 = Index Array(array=w1093, index=3) -> (element=w1162:waveform(dbl))
    n740 = Index Array(array=w1093, index=6) -> (element=w1159:waveform(dbl))
    n741 = Build Array(w1074, w1073) -> (→"APD Chart":waveform(dbl)[])
    n742 = Array Size(array=w1151) -> (size(s)=w1204:i32)
    n743 = call <vilib>:"Std Deviation and Variance.vi"("X"=w1086) -> ("standard deviation"=w1085:dbl)  [unwired: 1 in, 2 out]
    n744 = Add Array Elements(numeric array=w1086) -> (sum=w1088:u32)
    n745 = Add Array Elements(numeric array=w1151) -> (sum=w1214:u32)
    n746 = call <vilib>:"Std Deviation and Variance.vi"("X"=w1151) -> ("standard deviation"=w1150:dbl)  [unwired: 1 in, 2 out]
    n747 = Divide(x="T1 offset_x (mV)", y=1000.0) -> (x/y=w1163:dbl)
    n748 = Divide(x=w1085, y=w1084) -> (x/y=w1081:dbl)
    "Rate sigma (Hz) 2" <- w1081
    n749 = Multiply(x=w1084, y=w1204) -> (x*y=w1087:dbl)
    "Int. Time (s)" <- w1087
    n750 = Divide(x=w1088, y=w1087) -> (x/y=w1082:dbl)
    "APD 2 Rate (Hz)" <- w1082
    n751 = Divide(x=w1214, y=w1087) -> (x/y=w1148:dbl)
    "APD 1 Rate (Hz)" <- w1148
    n752 = Divide(x=w1150, y=w1084) -> (x/y=w1149:dbl)
    "Rate sigma (Hz)" <- w1149
    n753 = Divide(x=w1081, y=w1082) -> (x/y=→"Sigma/Mean 2":dbl)
    n754 = Divide(x=w1149, y=w1148) -> (x/y=→"Sigma/Mean":dbl)
    n755 = Divide(x="T2 offset_x (mV)", y=1000.0) -> (x/y=w1161:dbl)
    n756 = case shown="0, Default" "Calibration" {
      tunnel: "T1 alpha_x (nm/V)" -> [_ w2066 w2087]
      tunnel: "T1 kappa_x (pN/nm)" -> [_ _ w2077]
      tunnel: "T2 alpha_x (nm/V)" -> [_ w2065 w2085]
      tunnel: "T2 kappa_x (pN/nm)" -> [_ _ w2078]
      tunnel: w1162 -> [w2048 w2063 w2083]
      tunnel: w1159 -> [w2047 w2061 w2081]
      tunnel: [w2048 w2060 w2080] -> w985
      tunnel: [w2047 w2059 w2079] -> w986
      tunnel: ["T1 X (V)" ("Label.Text") "T1 X (nm)" ("Label.Text") "T1 X (pN)" ("Label.Text")] -> w1180
      tunnel: ["T2 X (V)" ("Label.Text") "T2 X (nm)" ("Label.Text") "T2 X (pN)" ("Label.Text")] -> w1179
      tunnel: ["Position (V)" ("Label.Text") "Position (nm)" ("Label.Text") "Force (pN)" ("Label.Text")] -> w1181
      tunnel: w1161 -> [_ w2051 w2070]
      tunnel: w1163 -> [_ w2054 w2072]
      tunnel: ["Mean (V)" ("Label.Text") "Mean (nm)" ("Label.Text") "Mean (pN)" ("Label.Text")] -> w1176
      tunnel: ["Difference (V)" ("Label.Text") "Difference (nm)" ("Label.Text") "Difference (pN)" ("Label.Text")] -> w1101
      frame 0, Default {
      }
      frame 1 {
        # "position"
        n757 = Unbundle By Name(w2063) -> ("Y"=w2067:dbl[])
        n758 = Unbundle By Name(w2061) -> ("Y"=w2052:dbl[])
        n759 = Subtract(x=w2067, y=w2054) -> (x-y=w2055:dbl[])
        n760 = Subtract(x=w2052, y=w2051) -> (x-y=w2053:dbl[])
        n761 = Multiply(x=w2053, y=w2065) -> (x*y=w2062:dbl[])
        n762 = Multiply(x=w2066, y=w2055) -> (x*y=w2064:dbl[])
        n763 = Bundle By Name(cluster=w2061, "Y"=w2062) -> (w2059:waveform(dbl))
        n764 = Bundle By Name(cluster=w2063, "Y"=w2064) -> (w2060:waveform(dbl))
      }
      frame 2 {
        # "force"
        n765 = Unbundle By Name(w2083) -> ("Y"=w2088:dbl[])
        n766 = Unbundle By Name(w2081) -> ("Y"=w2086:dbl[])
        n767 = Subtract(x=w2086, y=w2070) -> (x-y=w2071:dbl[])
        n768 = Subtract(x=w2088, y=w2072) -> (x-y=w2073:dbl[])
        n769 = Compound Arithmetic op=MULTIPLY(w2071, w2085, w2078) -> (w2082:dbl[])
        n770 = Compound Arithmetic op=MULTIPLY(w2077, w2087, w2073) -> (w2084:dbl[])
        n771 = Bundle By Name(cluster=w2081, "Y"=w2082) -> (w2079:waveform(dbl))
        n772 = Bundle By Name(cluster=w2083, "Y"=w2084) -> (w2080:waveform(dbl))
      }
    }
    n773 = feedback-in #17("Calibration") -> ()
    n774 = feedback #17(u16 1 ("Calibration")) -> (w1183:u16)
    n775 = Not Equal?(x=w1183, y="Calibration") -> (x != y?=w1139:bool)
    n776 = Unbundle By Name(w1162) -> ("Y"=w1165:dbl[])
    n777 = Unbundle By Name(w1159) -> ("Y"=w1168:dbl[])
    n778 = Subtract(x=w1165, y=w1163) -> (x-y=w1166:dbl[])
    n779 = Subtract(x=w1168, y=w1161) -> (x-y=w1167:dbl[])
    n780 = Multiply(x=w1167, y="T2 alpha_x (nm/V)") -> (x*y=w1158:dbl[])
    n781 = Multiply(x="T1 alpha_x (nm/V)", y=w1166) -> (x*y=w1157:dbl[])
    n782 = Multiply(x=w985, y=-1.0) -> (x*y=w983:waveform(dbl))
    n783 = Multiply(x=w986, y=1.0) -> (x*y=w1170:waveform(dbl))
    n784 = case shown="True" "Read Lateness and Rel Phase" {
      tunnel: w993 -> [w1623 w1645]
      tunnel: w992 -> [w1624 w1644]
      tunnel: [w1623 w1643] -> w1154
      tunnel: [w1624 w1642] -> w1153
      frame False {
      }
      frame True {
        n785 = xnode "Read/Write Control"("FPGA VI Reference In"=w1645, "error in"=w1644) -> ("FPGA VI Reference Out"=w1643:T20, "error out"=w1642:errorcluster, "GI Relative phase"=→"GI relative phase":i16, "Relative phase"=→"Relative phase (AI1)":i16, "AI Late Counter"=→"Late Counter (AI1)":u16, "GI Late Counter"=→"GI Late Counter":u16, "MCL Late Counter"=→"MCL Late Counter":u16, "MCL Relative Phase"=→"Relative Phase (MCL)":i16, "APD Acq Relative Phase"=→"APD Acq Relative Phase":i16, "APD 1 Gate Relative Phase"=→"APD 1 Gate Relative Phase":i16, "APD 2 Gate Relative Phase"=→"APD 2 Gate Relative Phase":i16, "APD Acq Late Counter"=→"APD Acq Late Counter":u16, "APD 1 Gate Late Counter"=→"APD 1 Gate Late Counter":u16, "APD 2 Gate Late Counter"=→"APD 2 Gate Late Counter":u16, "Green FB Relative Phase"=→"Relative phase (Green FB)":i16, "GI Relative phase 2"=→"GI relative phase 2":i16, "GI Late Counter 2"=→"GI Late Counter 2":u16, "Trap Pos FIFO Timeout"=→"Trap Pos FIFO Timeout":u16, "Trap AI FIFO Timeout"=→"Trap AI FIFO Timeout":u16)
      }
    }
    n786 = Subtract(x=w1158, y=w1157) -> (x-y=w1156:dbl[])
    n787 = Unbundle By Name(w986) -> ("Y"=w1126:dbl[])
    n788 = Unbundle By Name(w985) -> ("Y"=w1127:dbl[])
    n789 = Build Array(w983, w1170) -> (→"Force":waveform(dbl)[])
    n790 = Subtract(x=w1156, y="Offset (nm)") -> (x-y=w1124:dbl[])
    n791 = call <vilib>:"Mean.vi"("X"=w1126) -> ("mean"=w1105:dbl)  [unwired: 1 out]
    "T2 X" <- w1105
    n792 = Absolute Value(x=w1127) -> (abs(x)=w1128:dbl[])
    n793 = Absolute Value(x=w1126) -> (abs(x)=w1129:dbl[])